vi "overlay oblique sliced FL imgs to BF img-2 (SubVI).vi"(3 "calib(F)/monitor(T)":bool, 4 "config":T2={"Interpolation Type in"=0, "cam ofst"=100, "virtual slit center"=0.0, "virtual slit width ratio"=0.9999999999999999, "overlay x"=747, "overlay y"=485, "BF pixel size"=1.2000000000000002, "FL pixel size"=0.45500000000000007, "oblique angle"=45.0, "AOD scan speed ratio"=5.0, "Nx"=140.25, "y compensation"=0.0, "rotation [deg]"=0.0, "slice cut ofst"=0.0, "init pos mag"=1.035, "slice cut mag"=1.0000000000000004} {"slice cut mag" min=1e-05 format="%_4g"; "rotation [deg]" format="%.2f"; "y compensation" format="%_4g"; "Interpolation Type in" items=["Zero Order", "Bi-Linear", "Quadratic", "Cubic Spline"]}, 5 "scan pos in":T1={"img scan pos"=[[1141.3996899464964, 1144.6292217416394, 1145.0484398112017, 1144.8776472643426, 1144.706854717484, 1144.6758015271464, 1144.706854717484, 1144.5360621706257], [1022.3581473747339, 1025.5298857323035, 1025.995683587372, 1025.8248910405136, 1025.5764655178102, 1025.4522527564586, 1025.2357430127136, 1025.2823227982205], [896.297721197978, 899.2762397045561, 899.7575641547936, 899.6799311789489, 899.4625588465835, 899.4625588465835, 899.2762397045561, 899.1054471576975], [767.1104112719224, 770.314927997071, 770.4193012201512, 770.301126579143, 770.2700733888051, 770.115670025736, 769.8163517744233, 769.7257799692711], [635.1119250316625, 637.9998717330884, 638.1396110896089, 637.9377653524126, 637.766972805554, 637.9688185427505, 637.9998717330884, 637.6582866393713], [501.57285551519584, 504.63504511796236, 504.9145238310036, 504.72820468897606, 504.5884653324555, 504.5263589517796, 504.5574121421175, 504.06056109671096], [365.9790999047028, 368.6186210834256, 369.09994553366334, 368.5720412979188, 368.64967427376354, 368.6962540592704, 368.4633551317359, 368.02861046700525], [227.29210150110552, 230.08775122013805, 230.19471220907977, 230.36377957869726, 230.01615636463674, 229.93938597741248, 229.52189308509168, 229.82983722260929], [85.86897199329073, 88.30060931447332, 88.50331764029022, 88.27214388999688, 88.25661729482795, 88.10480169762036, 88.05994708935451, 87.93918468248482], [-58.202304579452054, -55.57313446417543, -55.619714249682296, -55.50067702005362, -55.51447843798161, -55.79913268274579, -56.13295447887834, -56.19074791645168], [-204.17127611728927, -201.5636707175252, -201.3928781706667, -201.37648898687726, -201.76465386610113, -201.71807408059428, -202.01307938880444, -202.01307938880444], [-350.91657741357477, -348.2615296396834, -348.1683700686696, -348.370215805866, -348.4012689962039, -348.52548175755555, -348.7739072802588, -348.8204870657657], [-496.3576447156677, -494.0752352258312, -493.59391077559354, -493.7181235369452, -493.9976022499864, -494.0752352258312, -494.1218150113381, -494.32366074853445], [-639.2368238148819, -636.5817760409902, -636.1936111617665, -636.5196696603145, -636.6283558264971, -636.5662494458215, -637.0320473008901, -637.2494196332556], [-775.4861467769537, -772.8190227623754, -772.7413897865306, -773.0182807337103, -772.8966557382201, -773.2529048384856, -773.3460644094994, -773.4711397594715], [-902.8025019851501, -900.3467121825935, -900.0715464126547, -900.1940339967655, -900.2716669726102, -900.5468327425489, -900.8047467400777, -900.7150375235459]], "g1 disp [um]"=0.9145564599592126, "z spacing [um]"=0.007201231968182777, "g2 disp [pixels]"=2047.850941796352, "scape scan pos "=[0.29732121750533475, 0.3339212016293517, 0.249904901396023, 0.1110940587916667, -0.0031212690815556675, -0.07248815619754172, -0.1281775480034735, -0.14486285062462914, -0.1685795718317721, -0.18878111894295188, -0.19064895657920522, -0.20565481091882423, -0.28052566429590736, -0.32633317813170115, -0.38861084538241164, -0.575312188665054, 0.30716242050115883, 0.33025082039455955, 0.22853341357629017, 0.10978710764331982, 0.0030795237131809555, -0.07652782338334116, -0.11905457942250673, -0.14273811841376213, -0.17025152735488258, -0.17933060977935283, -0.1928603907090043, -0.21629987985437663, -0.2902823061609209, -0.34034677717687495, -0.38567475447339, -0.5662170503296705, 0.3164555817378069, 0.3222592583359534, 0.2346539268164601, 0.08552555585918374, -0.016710992078617, -0.07869965293288726, -0.1295915385579094, -0.14070865127431448, -0.1611981343878737, -0.18317546524607017, -0.18317439485200931, -0.21692606037999748, -0.27968326416998684, -0.3331954744560679, -0.3859145227430294, -0.5788102364560431, 0.3222378504547357, 0.3253195149560384, 0.23405236535423973, 0.10453254319841006, 0.0013594004573304866, -0.06927483322674952, -0.12285661912678855, -0.16458272040840835, -0.17292109014274257, -0.18654506574975233, -0.1888025268241697, -0.20828476912643132, -0.27138663980402716, -0.3386683992893993, -0.38265945440386245, -0.5554617308058464, 0.3209801374331898, 0.31463805262241573, 0.22944753010429042, 0.10855080250299172, -0.012128635103946265, -0.07863542928923384, -0.12142871344956106, -0.15474579898882793, -0.1691672181712008, -0.18278584180790616, -0.1737956020904898, -0.19809354727269624, -0.2869362543265784, -0.33007099419232955, -0.37952319980545446, -0.5779453580548439, 0.3221297406545858, 0.3289492212165169, 0.22099783938762355, 0.11749929685203336, -0.010805628044686053, -0.07370626463883473, -0.1270108184771032, -0.14781285665644237, -0.15608914353524492, -0.1799407343940601, -0.1753123504747711, -0.18943084813791217, -0.2613495546950603, -0.3344103717151782, -0.37705594149510246, -0.5654560001523777, 0.3229507328992885, 0.33574622350316946, 0.2396333999877211, 0.1163668199356116, 0.007141669174259077, -0.07657492072202031, -0.1116067775468331, -0.14098909451826766, -0.15960966960151274, -0.16532343309854433, -0.1829421193407962, -0.19362251128035804, -0.27498744542486164, -0.32437863857651567, -0.39384079076392087, -0.5516393536144077, 0.30666361686878413, 0.32842365773261994, 0.24334766737900995, 0.11170097222419144, 0.007354677592376207, -0.06384258336773202, -0.122833070457449, -0.1424341265004693, -0.16672993089455398, -0.18028433088760595, -0.1743661221249442, -0.20595987322617793, -0.2873269481588033, -0.3277064937118232, -0.3803077986520869, -0.4931926267076228]}, 6 "image in":u16[][][](array[numeric])=array1x300x2304[691200 elements], 7 "BF image in":u16[][](array[numeric])=array1024x1280[1310720 elements]) -> (1 "overlaid image":u16[][](array[numeric]))   [LabVIEW 2024]
uses:
  Global variables/global for picoscope.vi
  <vilib>/vision/NI_Vision_Development_Module.lvlib
panel:
  out "Intensity Graph":u16[][](graph)
  in  "slice cut pos":path=path "F:/calibration/20210907-114245.calib"
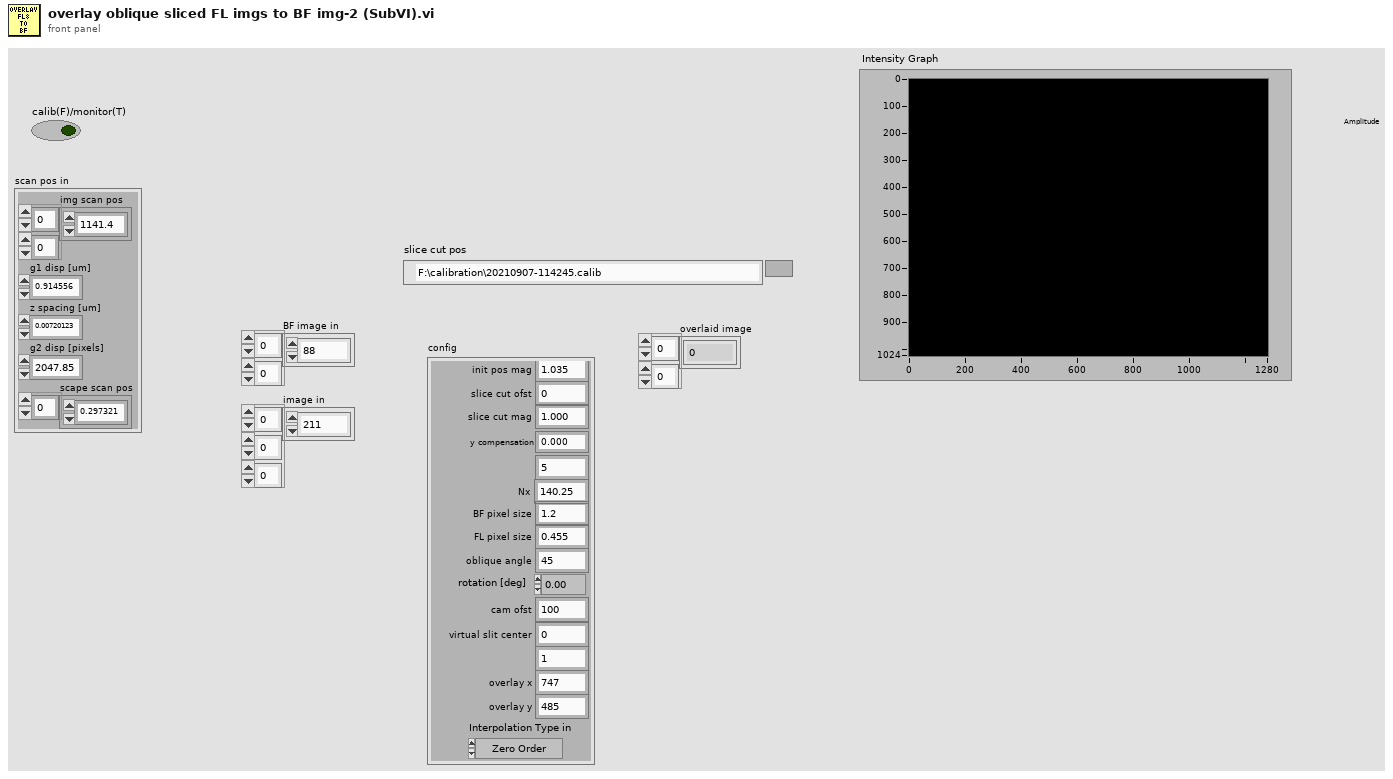
[diagram p1: front panel]
types:
  T1 = cluster{"img scan pos":dbl[][], "g1 disp [um]":dbl, "z spacing [um]":dbl, "g2 disp [pixels]":dbl, "scape scan pos ":dbl[]}
  T2 = cluster{"Interpolation Type in":u32, "cam ofst":u16, "virtual slit center":dbl, "virtual slit width ratio":dbl, "overlay x":i32, "overlay y":i32, "BF pixel size":dbl, "FL pixel size":dbl, "oblique angle":dbl, "AOD scan speed ratio":dbl, "Nx":dbl, "y compensation":dbl, "rotation [deg]":sgl, "slice cut ofst":dbl, "init pos mag":dbl, "slice cut mag":dbl}
  T3 = typedef "Image Type" = u32
  T4 = typedef "IMAQ Image.ctl" = refnum<image>
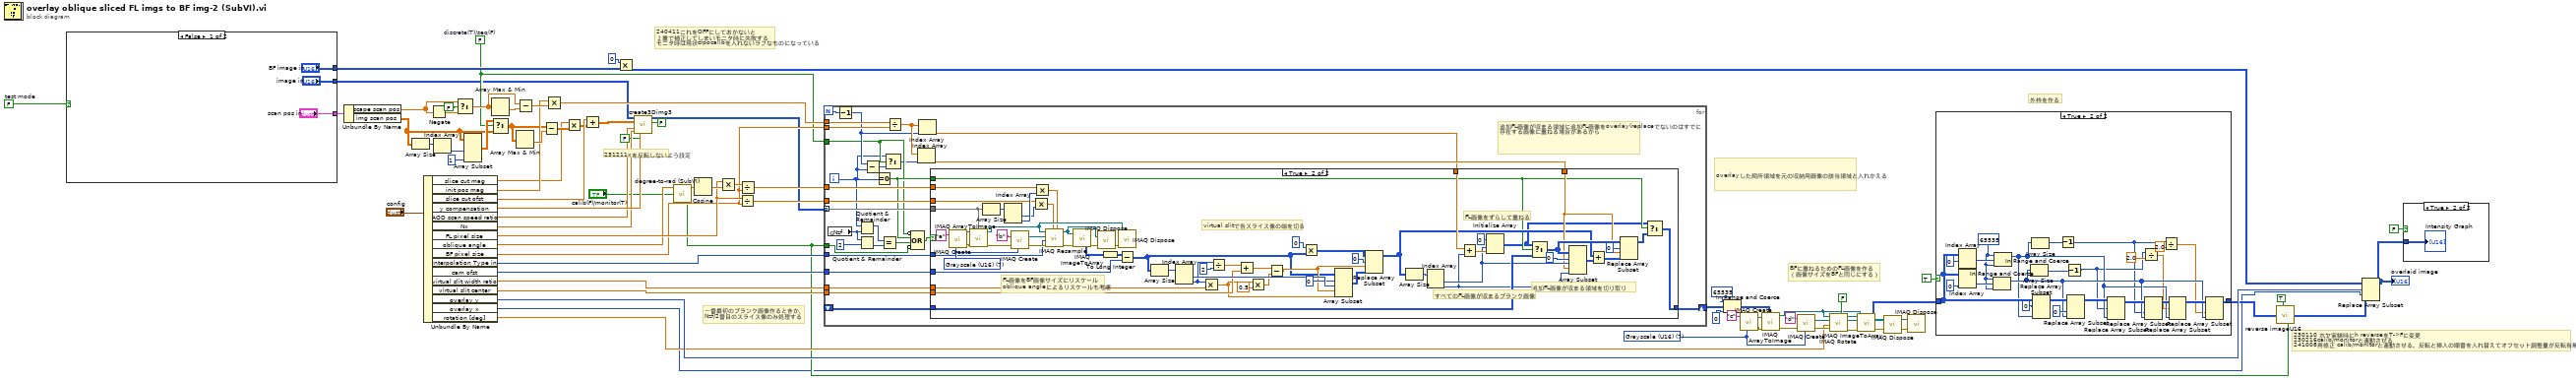
[diagram p0: block diagram]
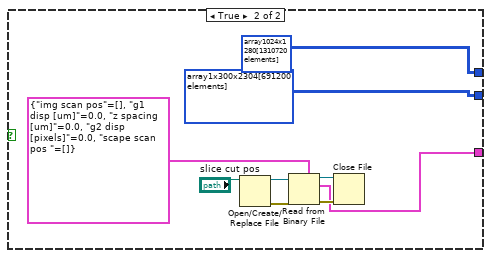
[diagram p4: hidden frame]
diagram:
  w13 = FALSE  # discrete(T)/seq(F)
  w33 = T3 7 items=["Grayscale (U8)", "Grayscale (I16)", "Grayscale (SGL)", "Complex (CSG)", "RGB (U32)", "HSL (U32)", "RGB (U64)", "Grayscale (U16)"] ("Image Type")
  w49 = FALSE  # test mode
  # "240411これをOFFにしておかないと\n２重で補正してしまいモニタ時に失敗する\nモニタ時は現状crpocalibを入れないラフなものになっている"
  # "231211xを反転しないよう設定"
  # "230110 ホヤ実験時にh reverseをT->Fに変更\n230216calib/monitorと連動させる\n241008再修正 calib/monitorと連動させる。反転と挿入の順番を入れ替えてオフセット調整量が反転有無で大きく変わらないように変更"
  # "外枠を作る"
  # "一番最初のブランク画像作るときか、\nNzf/2番目のスライス像のみ処理する"
  # "overlayした局所領域を元の収納用画像の該当領域と入れかえる"
  # "BFに重ねるためのFL画像を作る\n（画像サイズをBFと同じにする）"
  n1 = case shown="False" w49 {
    tunnel: ["BF image in" u16[][] array1024x1280[1310720 elements] ("img array")] -> w75
    tunnel: ["image in" u16[][][] array1x300x2304[691200 elements] ("Image")] -> w9
    tunnel: ["scan pos in" w81] -> w55
    frame False {
    }
    frame True {
      n2 = Open/Create/Replace File(file path (use dialog)="slice cut pos") -> (refnum out=w83:refnum<file>, error out=w82:errorcluster)  [unwired: 5 in, 1 out]
      n3 = Read from Binary File(5:T1 {"img scan pos"=[], "g1 disp [um]"=0.0, "z spacing [um]"=0.0, "g2 disp [pixels]"=0.0, "scape scan pos "=[]} ("output cluster 2"), 8:w82, 11:w83) -> (0:w87:errorcluster, 2:w81:T1, 3:w86:refnum<file>)  [unwired: 3 in, 1 out]
      n4 = Close File(refnum=w86, error in=w87) -> ()  [unwired: 2 out]
    }
  }
  n5 = Unbundle By Name(w55) -> ("scape scan pos"=w30:dbl[], "img scan pos"=w14:dbl[][])
  n6 = Array Size(array=w14) -> (size(s)=w60:i32[])
  n7 = Unbundle By Name("config") -> ("slice cut mag"=w21:dbl, "init pos mag"=w26:dbl, "slice cut ofst"=w23:dbl, "y compensation"=w58:dbl, "AOD scan speed ratio"=w56:dbl, "Nx"=w57:dbl, "FL pixel size"=w68:dbl, "oblique angle"=w67:dbl, "BF pixel size"=w52:dbl, "Interpolation Type in"=w66:u32, "cam ofst"=w65:u16, "virtual slit width ratio"=w64:dbl, "virtual slit center"=w63:dbl, "overlay y"=w62:i32, "overlay x"=w1:i32, "rotation [deg]"=w32:sgl)
  n8 = Negate(x=w30) -> (-x=w54:dbl[])
  n9 = Index Array(array=w60) -> (element=w59:i32)  [unwired: 1 in]
  n10 = Select(t=w30, s=FALSE ("Boolean"), f=w54) -> (s? t:f=w29:dbl[])
  n11 = Array Subset(array=w14, length (row)=w59, length (col)=1 ("length")) -> (w15:dbl[][])  [unwired: 2 in]
  n12 = Array Max & Min(array=w29) -> (min value=w28:dbl)  [unwired: 3 out]
  n13 = Select(t=w15, s=w13, f=w14) -> (s? t:f=w12:dbl[][])
  n14 = Array Max & Min(array=w12) -> (min value=w47:dbl)  [unwired: 3 out]
  n15 = Subtract(x=w29, y=w28) -> (x-y=w27:dbl[])
  n16 = Subtract(x=w12, y=w47) -> (x-y=w48:dbl[][])
  n17 = Multiply(x=w26, y=w27) -> (x*y=w25:dbl[])
  n18 = Multiply(x=w21, y=w48) -> (x*y=w22:dbl[][])
  n19 = Add(x=w23, y=w22) -> (x+y=w24:dbl[][])
  n20 = Multiply(x=u16 0 ("element"), y=w75) -> (x*y=w51:u16[][])
  n21 = call "create3Dimg3.vi"("input"=w9, "v comp"=w58, "x init pos"=w24, "AOD scan speed ratio"=w56, "cropcalib"=FALSE, "Nx"=w57, "reverse x"=FALSE) -> ("zyx"=w8:u16[][][])  [unwired: 7 in, 1 out]
  n22 = call "degree-to-rad (SubVI).vi"("oblique angle"=w67) -> ("Numeric"=w70:dbl)  [unwired: 10 in]
  n23 = Cosine(x=w70) -> (cos(x)=w71:dbl)
  n24 = Multiply(x=w68, y=w71) -> (x*y=w72:dbl)
  n25 = Divide(x=w68, y=w52) -> (x/y=w73:dbl)
  n26 = Divide(x=w72, y=w52) -> (x/y=w74:dbl)
  n27 = for {
    N -> [w106]
    tunnel: w8 -> [w115] mode=indexing
    tunnel: w73 -> [w114]
    tunnel: w74 -> [w113]
    shift-right: [w112] -> w19
    shift-left: _ -> [w111]
    tunnel: w64 -> [w109]
    tunnel: w63 -> [w110]
    tunnel: w66 -> [w108]
    tunnel: w65 -> [w107]
    tunnel: w25 -> [w105]
    tunnel: w52 -> [w104]
    tunnel: w13 -> [w91]
    tunnel: "calib(F)/monitor(T)" -> [w93]
    i -> [w90]
    # "追加FL画像が収まる領域に追加FL画像をoverlay(replaceでないのはすでに存在する画像に重ねる場合があるから"
    n28 = global read "global for picoscope.vi" "Nzf"() -> (w100:i32)
    n29 = Decrement(x=w106) -> (x-1=w92:i32)
    n30 = Quotient & Remainder(x=w90, y=w100) -> (x-y*floor(x/y)=w98:i32)  [unwired: 1 out]
    n31 = Quotient & Remainder(x=w100, y=2) -> (floor(x/y)=w97:i32)  [unwired: 1 out]
    n32 = Subtract(x=w92, y=w90) -> (x-y=w89:i32)
    n33 = Equal To 0?(x=w90) -> (x = 0?=w94:bool)
    n34 = Equal?(x=w98, y=w97) -> (x = y?=w95:bool)
    n35 = Select(t=w90, s=w91, f=w89) -> (s? t:f=w88:i32)
    n36 = Divide(x=w105, y=w104) -> (x/y=w102:dbl[])
    n37 = Compound Arithmetic op=OR(invert w91, w94, w95, invert w93) -> (w96:bool)
    n38 = Index Array(array=w102, index=w88) -> (element=w103:dbl)
    n39 = Index Array(array=w102, index=w92) -> (element=w101:dbl)
    n40 = case shown="True" w96 {
      tunnel: w115 -> [_ w165]
      tunnel: w114 -> [_ w162]
      tunnel: w113 -> [_ w161]
      tunnel: [w116 w117] -> w112
      tunnel: w94 -> [_ w120]
      tunnel: w111 -> [w116 w154]
      tunnel: w110 -> [_ w140]
      tunnel: w109 -> [_ w131]
      tunnel: w108 -> [_ w127]
      tunnel: w107 -> [_ w126]
      tunnel: w103 -> [_ w125]
      tunnel: w101 -> [_ w124]
      frame False {
      }
      frame True {
        w158 = T3 7 items=["Grayscale (U8)", "Grayscale (I16)", "Grayscale (SGL)", "Complex (CSG)", "RGB (U32)", "HSL (U32)", "RGB (U64)", "Grayscale (U16)"] ("Image Type")
        # "追加FL画像が収まる領域を切り取り"
        # "すべてのFL画像が収まるブランク画像"
        # "FL画像をずらして重ねる"
        # "virtual slitで各スライス像の端を切る"
        # "FL画像をBF画像サイズにリスケール\noblique angleによるリスケールも考慮"
        n41 = call "IMAQ Create"("Image Name"="a", "Image Type"=w158) -> ("New Image"=w174:T4, "error out"=w168:errorcluster)  [unwired: 3 in]
        n42 = call "IMAQ ArrayToImage"("Image Pixels (U16)"=w165, "error in (no error)"=w168, "Image"=w174) -> ("error out"=w167:errorcluster, "Image Out"=w171:T4)  [unwired: 7 in]
        n43 = Array Size(array=w165) -> (size(s)=w166:i32[])
        n44 = Index Array(array=w166) -> (element #1=w163:i32, element #2=w164:i32)  [unwired: 2 in]
        n45 = call "IMAQ Create"("Image Name"="b", "Image Type"=w158, "error in (no error)"=w167) -> ("New Image"=w173:T4, "error out"=w169:errorcluster)  [unwired: 2 in]
        n46 = Multiply(x=w162, y=w163) -> (x*y=w160:dbl)
        n47 = Multiply(x=w161, y=w164) -> (x*y=w159:dbl)
        n48 = call "IMAQ Resample"("X Resolution"=w159, "Y Resolution"=w160, "error in (no error)"=w169, "Interpolation Type"=w127, "Image Dst"=w173, "Image Src"=w171) -> ("error out"=w170:errorcluster, "Image Dst Out"=w172:T4)  [unwired: 4 in]
        n49 = call "IMAQ ImageToArray"("error in (no error)"=w170, "Image"=w172) -> ("Image Pixels (U16)"=w129:u16[][], "error out"=w177:errorcluster)  [unwired: 2 in, 3 out]
        n50 = call "IMAQ Dispose"("Image"=w172, "error in (no error)"=w177) -> ("error out"=w123:errorcluster)  [unwired: 4 in]
        n51 = To Long Integer(number=w129) -> (32bit integer=w121:i32[][])
        n52 = call "IMAQ Dispose"("Image"=w171, "error in (no error)"=w123) -> ()  [unwired: 4 in, 1 out]
        n53 = Subtract(x=w121, y=w126) -> (x-y=w128:i32[][])
        n54 = Array Size(array=w128) -> (size(s)=w146:i32[])
        n55 = Index Array(array=w146) -> (element #1=w145:i32, element #2=w132:i32)  [unwired: 2 in]
        n56 = Multiply(x=w132, y=w131) -> (x*y=w130:dbl)
        n57 = Divide(x=w132, y=2) -> (x/y=w141:dbl)
        n58 = Add(x=w141, y=w140) -> (x+y=w139:dbl)
        n59 = Multiply(x=w130, y=0.5) -> (x*y=w138:dbl)
        n60 = Subtract(x=w139, y=w138) -> (x-y=w133:dbl)
        n61 = Multiply(x=u16 0, y=w128) -> (x*y=w136:i32[][])
        n62 = Array Subset(array=w128, index (row)=0 ("index"), length (row)=w145, index (col)=w133, length (col)=w130) -> (w135:i32[][])
        n63 = Replace Array Subset(array=w136, new element=w135, index (row)=0, index (col)=w133) -> (w122:i32[][])
        n64 = Array Size(array=w122) -> (size(s)=w157:i32[])
        n65 = Index Array(array=w157) -> (element #1=w152:i32, element #2=w151:i32)  [unwired: 2 in]
        n66 = Add(x=w124, y=w151) -> (x+y=w155:dbl)
        n67 = Initialize Array(0 ("element"), w152, w155) -> (w119:i32[][])
        n68 = Select(t=w119, s=w120, f=w154) -> (s? t:f=w153:i32[][])
        n69 = Array Subset(array=w153, index (row)=0 ("disabled index (col)"), length (row)=w152, index (col)=w125, length (col)=w151) -> (w149:i32[][])
        n70 = Add(x=w122, y=w149) -> (x+y=w148:i32[][])
        n71 = Replace Array Subset(array=w153, new element=w148, index (row)=0 ("disabled index (col)"), index (col)=w125) -> (w118:i32[][])
        n72 = Select(t=w119, s=w120, f=w118) -> (s? t:f=w117:i32[][])
      }
    }
  }
  n73 = In Range and Coerce(upper limit=65535, x=w19, lower limit=0) -> (coerced(x)=w18:i32[][])  [unwired: 1 out]
  n74 = call "IMAQ Create"("Image Name"="c", "Image Type"=w33) -> ("New Image"=w43:T4, "error out"=w42:errorcluster)  [unwired: 3 in]
  n75 = call "IMAQ ArrayToImage"("Image Pixels (U16)"=w18, "error in (no error)"=w42, "Image"=w43) -> ("error out"=w39:errorcluster, "Image Out"=w34:T4)  [unwired: 7 in]
  n76 = call "IMAQ Create"("Image Name"="d", "Image Type"=w33, "error in (no error)"=w39) -> ("New Image"=w41:T4, "error out"=w40:errorcluster)  [unwired: 2 in]
  n77 = call "IMAQ Rotate"("Maintain Size"=FALSE, "error in (no error)"=w40, "Angle (degrees)"=w32, "Image Dst"=w41, "Image Src"=w34) -> ("error out"=w36:errorcluster, "Image Dst Out"=w35:T4)  [unwired: 5 in]
  n78 = call "IMAQ ImageToArray"("error in (no error)"=w36, "Image"=w35) -> ("Image Pixels (U16)"=w11:u16[][], "error out"=w37:errorcluster)  [unwired: 2 in, 3 out]
  n79 = call "IMAQ Dispose"("Image"=w35, "error in (no error)"=w37) -> ("error out"=w38:errorcluster)  [unwired: 4 in]
  n80 = call "IMAQ Dispose"("Image"=w34, "error in (no error)"=w38) -> ()  [unwired: 4 in, 1 out]
  n81 = case shown="True" TRUE {
    tunnel: w11 -> [w178 w200]
    tunnel: [w178 w187] -> w3
    frame False {
    }
    frame True {
      w198 = 65535
      n82 = Index Array(array=w200, index (row)=0) -> (element=w202:u16[])  [unwired: 1 in]
      n83 = Index Array(array=w200, index (col)=0 ("disabled index (col)")) -> (element=w199:u16[])  [unwired: 1 in]
      n84 = In Range and Coerce(upper limit=w198, x=w199, lower limit=w198) -> (coerced(x)=w186:i32[])  [unwired: 1 out]
      n85 = In Range and Coerce(upper limit=w198, x=w202, lower limit=w198) -> (coerced(x)=w185:i32[])  [unwired: 1 out]
      n86 = Array Size(array=w186) -> (size(s)=w191:i32)
      n87 = Array Size(array=w185) -> (size(s)=w193:i32)
      n88 = Replace Array Subset(array=w200, new element=w185, index (row)=0) -> (w196:u16[][])  [unwired: 1 in]
      n89 = Decrement(x=w193) -> (x-1=w180:i32)
      n90 = Decrement(x=w191) -> (x-1=w182:i32)
      n91 = Replace Array Subset(array=w196, new element=w186, index (col)=0) -> (w195:u16[][])  [unwired: 1 in]
      n92 = Replace Array Subset(array=w195, new element=w185, index (row)=w182) -> (w194:u16[][])  [unwired: 1 in]
      n93 = Divide(x=w182, y=2.0) -> (x/y=w181:dbl)
      n94 = Replace Array Subset(array=w194, new element=w186, index (col)=w180) -> (w188:u16[][])  [unwired: 1 in]
      n95 = Divide(x=w180, y=2.0) -> (x/y=w179:dbl)
      n96 = Replace Array Subset(array=w188, new element=w185, index (row)=w181) -> (w189:u16[][])  [unwired: 1 in]
      n97 = Replace Array Subset(array=w189, new element=w186, index (col)=w179) -> (w187:u16[][])  [unwired: 1 in]
    }
  }
  n98 = call "reverse imageU16.vi"("output array in"=w3, "reverse v"=TRUE, "reverse h"="calib(F)/monitor(T)") -> ("output array out"=w2:u16[][])
  n99 = Replace Array Subset(array=w51, new element=w2, index (row)=w62, index (col)=w1) -> (w4:u16[][])
  "overlaid image" <- w4
  n100 = case shown="True" FALSE {
    tunnel: w4 -> [_ w203]
    frame False {
    }
    frame True {
      "Intensity Graph" <- w203
    }
  }
